vi "Dresden R2R Sputter 03.02.2018 IY24.vi"() -> ()   [LabVIEW 2009] (continued)
                      n13368 = Greater?(x=w19990, y=50) -> (0:w19991:bool)
                      n13369 = local read "Cnt_Right_slow_di"() -> (w19993:bool)
                      n13370 = case shown="True" w19991 {
                        frame #0 {
                        }
                        frame #1 {
                          n13371 = local write "Semi"(TRUE ("Semi")) -> ()
                          n13372 = local write "Error Message"("\nPlease check Left Slow Sensor\nconnections." ("Error Message")) -> ()
                        }
                      }
                      n13373 = case shown="True" w19993 {
                        tunnel: [TRUE ("Cnt_Left_slow_do") FALSE ("Cnt_Left_slow_do")] -> w19989
                        frame #0 {
                        }
                        frame #1 {
                          n13374 = local write "Cnt_Right_slow_do"(FALSE ("Cnt_Left_slow_do")) -> ()
                          n13375 = Wait Until Next ms Multiple(millisecond multiple=u32 200) -> ()  [unwired: 1 out]
                        }
                      }
                      n13376 = local read "Semi"() -> (w19988:bool)
                      n13377 = Or(x=w19989, y=w19988) -> (x .or. y?=w19987:bool)
                    }
                  }
                  frame #2 {
                    n13378 = while {
                      i -> [w20003]
                      stop <- w20000 stop-if-true
                      n13379 = Greater?(x=w20003, y=50) -> (0:w20004:bool)
                      n13380 = local read "Cnt_Right_limit_di"() -> (w20006:bool)
                      n13381 = case shown="True" w20004 {
                        frame #0 {
                        }
                        frame #1 {
                          n13382 = local write "Semi"(TRUE ("Semi")) -> ()
                          n13383 = local write "Error Message"("\nPlease check Left Limit Sensor\n connections." ("Error Message")) -> ()
                        }
                      }
                      n13384 = case shown="True" w20006 {
                        tunnel: [TRUE ("Cnt_Left_slow_do") FALSE ("Cnt_Left_slow_do")] -> w20002
                        frame #0 {
                        }
                        frame #1 {
                          n13385 = local write "Cnt_Right_limit_do"(FALSE ("Cnt_Left_slow_do")) -> ()
                          n13386 = Wait Until Next ms Multiple(millisecond multiple=u32 200) -> ()  [unwired: 1 out]
                        }
                      }
                      n13387 = local read "Semi"() -> (w20001:bool)
                      n13388 = Or(x=w20002, y=w20001) -> (x .or. y?=w20000:bool)
                    }
                  }
                  frame #3 {
                    n13389 = local read "Semi"() -> (w20013:bool)
                    n13390 = case shown="False" w20013 {
                      frame #0 {
                        n13391 = local write "CH1_2trns_12"(TRUE ("CH1_2trns_11")) -> ()
                        n13392 = Wait (ms)(milliseconds to wait=u32 500) -> ()  [unwired: 1 out]
                      }
                      frame #1 {
                      }
                    }
                  }
                }
              }
              frame #1 {
              }
            }
          }
          frame #17 {
            # "SET CASSETTE SERVO  SPEED 100"
            n13393 = local read "Semi"() -> (w20016:bool)
            n13394 = case shown="False" w20016 {
              frame #0 {
                n13395 = stacked-sequence {
                  frame #0 {
                    n13396 = while {
                      i -> [w20023]
                      stop <- w20019 stop-if-true
                      n13397 = local read "Ch2_Right_slow_di"() -> (w20017:bool)
                      n13398 = Greater?(x=w20023, y=1500) -> (0:w20022:bool)
                      n13399 = case shown="True" w20022 {
                        frame #0 {
                        }
                        frame #1 {
                          n13400 = local write "Semi"(TRUE ("Semi")) -> ()
                          n13401 = local write "Error Message"("Transfer process was cancelled.\nPlease check Casette & Sensor\nconnections." ("Error Message")) -> ()
                        }
                      }
                      n13402 = case shown="False" w20017 {
                        tunnel: [FALSE TRUE] -> w20020
                        frame #0 {
                          n13403 = Wait Until Next ms Multiple(millisecond multiple=u32 200) -> ()  [unwired: 1 out]
                        }
                        frame #1 {
                        }
                      }
                      n13404 = local read "Semi"() -> (w20018:bool)
                      n13405 = Or(x=w20020, y=w20018) -> (x .or. y?=w20019:bool)
                    }
                  }
                  frame #1 {
                    n13406 = disable-structure shown="Disabled" {
                      frame #0 {
                        n13407 = while {
                          i -> [w20038]
                          stop <- w20034 stop-if-true
                          n13408 = local read "Counter_read_data"() -> (w20031:i16)
                          n13409 = Greater?(x=w20038, y=5000) -> (0:w20037:bool)
                          n13410 = case shown="True" w20037 {
                            frame #0 {
                            }
                            frame #1 {
                              n13411 = local write "Semi"(TRUE ("Semi")) -> ()
                            }
                          }
                          n13412 = In Range and Coerce(upper limit=i16 1990, x=w20031, lower limit=i16 1980 ("upper limit")) -> (In Range?=w20029:bool)  [unwired: 1 out]
                          n13413 = case shown="True" w20029 {
                            tunnel: [FALSE TRUE] -> w20035
                            frame #0 {
                              n13414 = Wait Until Next ms Multiple(millisecond multiple=u32 200) -> ()  [unwired: 1 out]
                            }
                            frame #1 {
                            }
                          }
                          n13415 = local read "Semi"() -> (w20033:bool)
                          n13416 = Or(x=w20035, y=w20033) -> (x .or. y?=w20034:bool)
                        }
                      }
                      frame #1 {
                      }
                    }
                  }
                  frame #2 {
                    n13417 = local read "Semi"() -> (w20043:bool)
                    n13418 = case shown="False" w20043 {
                      frame #0 {
                        n13419 = local write "Cassette_servo_speed_value"(u16 100 ("Cassette_servo_speed_value")) -> ()
                      }
                      frame #1 {
                      }
                    }
                  }
                  frame #3 {
                    n13420 = local read "Semi"() -> (w20045:bool)
                    n13421 = case shown="False" w20045 {
                      frame #0 {
                        n13422 = Wait (ms)(milliseconds to wait=u32 200 ("millisecond multiple")) -> ()  [unwired: 1 out]
                      }
                      frame #1 {
                      }
                    }
                  }
                  frame #4 {
                    n13423 = local read "Semi"() -> (w20047:bool)
                    n13424 = case shown="False" w20047 {
                      frame #0 {
                        n13425 = local write "Cassette_servo_speed_auto_set"(TRUE ("Cassette_servo_speed_auto_set")) -> ()
                      }
                      frame #1 {
                      }
                    }
                  }
                  frame #5 {
                    n13426 = local read "Semi"() -> (w20049:bool)
                    n13427 = case shown="False" w20049 {
                      frame #0 {
                        n13428 = Wait (ms)(milliseconds to wait=u32 200 ("millisecond multiple")) -> ()  [unwired: 1 out]
                      }
                      frame #1 {
                      }
                    }
                  }
                  frame #6 {
                    n13429 = while {
                      i -> [w20054]
                      stop <- w20051 stop-if-true
                      n13430 = Greater?(x=w20054, y=50) -> (0:w20055:bool)
                      n13431 = local read "Cnt_Right_slow_di"() -> (w20057:bool)
                      n13432 = case shown="True" w20055 {
                        frame #0 {
                        }
                        frame #1 {
                          n13433 = local write "Semi"(TRUE ("Semi")) -> ()
                          n13434 = local write "Error Message"("\nPlease check connections." ("Error Message")) -> ()
                        }
                      }
                      n13435 = case shown="False" w20057 {
                        tunnel: [FALSE ("Cnt_Left_slow_do") TRUE ("Cnt_Left_slow_do")] -> w20053
                        frame #0 {
                          n13436 = local write "Cnt_Right_slow_do"(TRUE ("Cnt_Left_slow_do")) -> ()
                          n13437 = Wait Until Next ms Multiple(millisecond multiple=u32 200) -> ()  [unwired: 1 out]
                        }
                        frame #1 {
                        }
                      }
                      n13438 = local read "Semi"() -> (w20052:bool)
                      n13439 = Or(x=w20053, y=w20052) -> (x .or. y?=w20051:bool)
                    }
                  }
                  frame #7 {
                    n13440 = local read "Semi"() -> (w20064:bool)
                    n13441 = case shown="False" w20064 {
                      frame #0 {
                        n13442 = local write "CH1_2trns_12"(TRUE ("CH1_2trns_11")) -> ()
                        n13443 = Wait (ms)(milliseconds to wait=u32 500) -> ()  [unwired: 1 out]
                      }
                      frame #1 {
                      }
                    }
                  }
                }
              }
              frame #1 {
              }
            }
          }
          frame #18 {
            # "CASETTE STOP AND FIX"
            n13444 = local read "Semi"() -> (w20067:bool)
            n13445 = case shown="False" w20067 {
              frame #0 {
                n13446 = stacked-sequence {
                  frame #0 {
                    # "Center Casette stop"
                    n13447 = local read "Semi"() -> (w20068:bool)
                    n13448 = case shown="False" w20068 {
                      frame #0 {
                        n13449 = stacked-sequence {
                          frame #0 {
                            n13450 = while {
                              i -> [w20075]
                              stop <- w20070 stop-if-true
                              n13451 = local read "Ch2_Right_limit_di"() -> (w20069:bool)
                              n13452 = Greater?(x=w20075, y=600) -> (0:w20073:bool)
                              n13453 = case shown="True" w20073 {
                                frame #0 {
                                }
                                frame #1 {
                                n13454 = local write "Semi"(TRUE ("Semi")) -> ()
                                n13455 = local write "Error Message"("Transfer process was cancelled.\nPlease check Casette connections." ("Error Message")) -> ()
                                }
                              }
                              n13456 = case shown="False" w20069 {
                                tunnel: [FALSE TRUE] -> w20072
                                frame #0 {
                                n13457 = Wait Until Next ms Multiple(millisecond multiple=u32 200) -> ()  [unwired: 1 out]
                                }
                                frame #1 {
                                }
                              }
                              n13458 = local read "Semi"() -> (w20071:bool)
                              n13459 = Or(x=w20072, y=w20071) -> (x .or. y?=w20070:bool)
                            }
                          }
                          frame #1 {
                            n13460 = disable-structure shown="Disabled" {
                              frame #0 {
                                n13461 = while {
                                i -> [w20090]
                                stop <- w20085 stop-if-true
                                n13462 = local read "Counter_read_data"() -> (w20082:i16)
                                n13463 = Greater?(x=w20090, y=5000) -> (0:w20088:bool)
                                n13464 = case shown="True" w20088 {
                                frame #0 {
                                }
                                frame #1 {
                                n13465 = local write "Semi"(TRUE ("Semi")) -> ()
                                n13466 = local write "Error Message"("Transfer process was cancelled.\nPlease check Casette connections." ("Error Message")) -> ()
                                }
                                }
                                n13467 = In Range and Coerce(upper limit=i16 2209, x=w20082, lower limit=i16 2199 ("upper limit")) -> (In Range?=w20081:bool)  [unwired: 1 out]
                                n13468 = case shown="True" w20081 {
                                tunnel: [FALSE TRUE] -> w20087
                                frame #0 {
                                }
                                frame #1 {
                                n13469 = Wait Until Next ms Multiple(millisecond multiple=u32 500) -> ()  [unwired: 1 out]
                                }
                                }
                                n13470 = local read "Semi"() -> (w20086:bool)
                                n13471 = Or(x=w20087, y=w20086) -> (x .or. y?=w20085:bool)
                                }
                              }
                              frame #1 {
                              }
                            }
                          }
                          frame #2 {
                            n13472 = while {
                              i -> [w20102]
                              stop <- w20097 stop-if-true
                              n13473 = local read "Casette_servo_start/stop_di"() -> (w20096:bool)
                              n13474 = Greater?(x=w20102, y=50) -> (0:w20100:bool)
                              n13475 = case shown="True" w20100 {
                                frame #0 {
                                }
                                frame #1 {
                                n13476 = local write "Semi"(TRUE ("Semi")) -> ()
                                n13477 = local write "Error Message"("Transfer process was cancelled.\nPlease check Casette connections." ("Error Message")) -> ()
                                }
                              }
                              n13478 = case shown="True" w20096 {
                                tunnel: [TRUE FALSE] -> w20099
                                frame #0 {
                                }
                                frame #1 {
                                n13479 = Wait Until Next ms Multiple(millisecond multiple=u32 200) -> ()  [unwired: 1 out]
                                n13480 = local write "Casette_servo_start/stop_do"(FALSE ("Casette_servo_start/stop_di")) -> ()
                                }
                              }
                              n13481 = local read "Semi"() -> (w20098:bool)
                              n13482 = Or(x=w20099, y=w20098) -> (x .or. y?=w20097:bool)
                            }
                          }
                          frame #3 {
                            n13483 = local read "Semi"() -> (w20109:bool)
                            n13484 = case shown="False" w20109 {
                              frame #0 {
                                n13485 = Wait (ms)(milliseconds to wait=u32 200) -> ()  [unwired: 1 out]
                              }
                              frame #1 {
                              }
                            }
                          }
                          frame #4 {
                            n13486 = local read "Semi"() -> (w20111:bool)
                            n13487 = case shown="False" w20111 {
                              frame #0 {
                                n13488 = local write "Cassette_servo_speed_value"(u16 0 ("Cassette_servo_speed_value")) -> ()
                              }
                              frame #1 {
                              }
                            }
                          }
                          frame #5 {
                            n13489 = local read "Semi"() -> (w20113:bool)
                            n13490 = case shown="False" w20113 {
                              frame #0 {
                                n13491 = Wait (ms)(milliseconds to wait=u32 200) -> ()  [unwired: 1 out]
                              }
                              frame #1 {
                              }
                            }
                          }
                          frame #6 {
                            n13492 = local read "Semi"() -> (w20115:bool)
                            n13493 = case shown="False" w20115 {
                              frame #0 {
                                n13494 = local write "Cassette_servo_speed_auto_set"(TRUE ("Cassette_servo_speed_auto_set")) -> ()
                              }
                              frame #1 {
                              }
                            }
                          }
                          frame #7 {
                            n13495 = local read "Semi"() -> (w20117:bool)
                            n13496 = case shown="False" w20117 {
                              frame #0 {
                                n13497 = Wait (ms)(milliseconds to wait=u32 200) -> ()  [unwired: 1 out]
                              }
                              frame #1 {
                              }
                            }
                          }
                          frame #8 {
                            n13498 = local read "Semi"() -> (w20119:bool)
                            n13499 = case shown="False" w20119 {
                              frame #0 {
                                n13500 = local write "CH1_2trns_13"(TRUE ("CH1_2trns_9")) -> ()
                                n13501 = Wait (ms)(milliseconds to wait=u32 500) -> ()  [unwired: 1 out]
                              }
                              frame #1 {
                              }
                            }
                          }
                        }
                      }
                      frame #1 {
                      }
                    }
                  }
                  frame #1 {
                    # "CASETTE FIX DOWN CH2"
                    n13502 = local read "Semi"() -> (w20122:bool)
                    n13503 = case shown="False" w20122 {
                      frame #0 {
                        n13504 = stacked-sequence {
                          frame #0 {
                            n13505 = local read "Semi"() -> (w20123:bool)
                            n13506 = case shown="False" w20123 {
                              frame #0 {
                                n13507 = while {
                                i -> [w20130]
                                stop <- w20125 stop-if-true
                                n13508 = Greater?(x=w20130, y=50) -> (0:w20128:bool)
                                n13509 = local read "Ch2_Cst_fix_down_di"() -> (w20124:bool)
                                n13510 = case shown="True" w20128 {
                                frame #0 {
                                }
                                frame #1 {
                                n13511 = local write "Semi"(TRUE ("Semi")) -> ()
                                n13512 = local write "Error Message"("Up/Down positions could not reach\nthe down position.\nPlease check connections." ("Error Message")) -> ()
                                }
                                }
                                n13513 = case shown="False" w20124 {
                                tunnel: [FALSE TRUE] -> w20127
                                frame #0 {
                                n13514 = Wait Until Next ms Multiple(millisecond multiple=u32 200) -> ()  [unwired: 1 out]
                                n13515 = local write "Ch2_Cst_fix_do"(TRUE ("Ch1_pet_cool_up_do")) -> ()
                                }
                                frame #1 {
                                }
                                }
                                n13516 = local read "Semi"() -> (w20126:bool)
                                n13517 = Or(x=w20127, y=w20126) -> (x .or. y?=w20125:bool)
                                }
                              }
                              frame #1 {
                              }
                            }
                          }
                          frame #1 {
                            n13518 = local read "Semi"() -> (w20137:bool)
                            n13519 = case shown="False" w20137 {
                              frame #0 {
                                n13520 = local write "CH1_2trns_14"(TRUE ("CH1_2trns_9")) -> ()
                                n13521 = Wait (ms)(milliseconds to wait=u32 500) -> ()  [unwired: 1 out]
                              }
                              frame #1 {
                              }
                            }
                          }
                        }
                      }
                      frame #1 {
                      }
                    }
                  }
                  frame #2 {
                    n13522 = local read "Semi"() -> (w20140:bool)
                    n13523 = case shown="False" w20140 {
                      frame #0 {
                        n13524 = stacked-sequence {
                          frame #0 {
                            n13525 = local read "Semi"() -> (w20141:bool)
                            n13526 = case shown="False" w20141 {
                              frame #0 {
                                n13527 = while {
                                i -> [w20148]
                                stop <- w20143 stop-if-true
                                n13528 = Greater?(x=w20148, y=50) -> (0:w20146:bool)
                                n13529 = local read "Ch2_trns_gv_bp2_di"() -> (w20142:bool)
                                n13530 = case shown="True" w20146 {
                                frame #0 {
                                }
                                frame #1 {
                                n13531 = local write "Semi"(TRUE ("Semi")) -> ()
                                n13532 = local write "Error Message"("Transfer process was cancelled.\nPlease check CH1-Trns-GV connections." ("Error Message")) -> ()
                                }
                                }
                                n13533 = case shown="True" w20142 {
                                tunnel: [TRUE FALSE] -> w20145
                                frame #0 {
                                }
                                frame #1 {
                                n13534 = Wait Until Next ms Multiple(millisecond multiple=u32 200) -> ()  [unwired: 1 out]
                                n13535 = local write "Ch2_trns_gv_bp2_do"(FALSE ("Ch1_pet_cool_up_do")) -> ()
                                }
                                }
                                n13536 = local read "Semi"() -> (w20144:bool)
                                n13537 = Or(x=w20145, y=w20144) -> (x .or. y?=w20143:bool)
                                }
                              }
                              frame #1 {
                              }
                            }
                          }
                          frame #1 {
                            n13538 = local read "Semi"() -> (w20155:bool)
                            n13539 = case shown="False" w20155 {
                              frame #0 {
                                n13540 = Wait (ms)(milliseconds to wait=u32 500) -> ()  [unwired: 1 out]
                              }
                              frame #1 {
                              }
                            }
                          }
                          frame #2 {
                            n13541 = local read "Semi"() -> (w20157:bool)
                            n13542 = case shown="False" w20157 {
                              frame #0 {
                                n13543 = while {
                                i -> [w20164]
                                stop <- w20159 stop-if-true
                                n13544 = Greater?(x=w20164, y=50) -> (0:w20162:bool)
                                n13545 = local read "Ch3_Trns_gv_bp_di"() -> (w20158:bool)
                                n13546 = case shown="True" w20162 {
                                frame #0 {
                                }
                                frame #1 {
                                n13547 = local write "Semi"(TRUE ("Semi")) -> ()
                                n13548 = local write "Error Message"("Transfer process was cancelled.\nPlease check CH1-Trns-GV connections." ("Error Message")) -> ()
                                }
                                }
                                n13549 = case shown="True" w20158 {
                                tunnel: [TRUE FALSE] -> w20161
                                frame #0 {
                                }
                                frame #1 {
                                n13550 = local write "Ch3_Trns_gv_bp_do"(FALSE ("Ch1_pet_cool_up_do")) -> ()
                                n13551 = Wait Until Next ms Multiple(millisecond multiple=u32 200) -> ()  [unwired: 1 out]
                                }
                                }
                                n13552 = local read "Semi"() -> (w20160:bool)
                                n13553 = Or(x=w20161, y=w20160) -> (x .or. y?=w20159:bool)
                                }
                              }
                              frame #1 {
                              }
                            }
                          }
                          frame #3 {
                            n13554 = local read "Semi"() -> (w20171:bool)
                            n13555 = case shown="False" w20171 {
                              frame #0 {
                                n13556 = Wait (ms)(milliseconds to wait=u32 500) -> ()  [unwired: 1 out]
                              }
                              frame #1 {
                              }
                            }
                          }
                        }
                      }
                      frame #1 {
                      }
                    }
                  }
                  frame #3 {
                    n13557 = local read "Semi"() -> (w20173:bool)
                    n13558 = case shown="False" w20173 {
                      frame #0 {
                        n13559 = stacked-sequence {
                          frame #0 {
                            n13560 = local read "Semi"() -> (w20174:bool)
                            n13561 = case shown="False" w20174 {
                              frame #0 {
                                n13562 = local write "Ch2_Trns_gv_open_do"(FALSE ("Ch1_pet_cool_up_do")) -> ()
                              }
                              frame #1 {
                              }
                            }
                          }
                          frame #1 {
                            n13563 = local read "Semi"() -> (w20176:bool)
                            n13564 = case shown="False" w20176 {
                              frame #0 {
                                n13565 = while {
                                i -> [w20183]
                                stop <- w20178 stop-if-true
                                n13566 = Greater?(x=w20183, y=500) -> (0:w20181:bool)
                                n13567 = local read "Ch2_Trns_gv_close_di"() -> (w20177:bool)
                                n13568 = case shown="True" w20181 {
                                frame #0 {
                                }
                                frame #1 {
                                n13569 = local write "Semi"(TRUE ("Semi")) -> ()
                                n13570 = local write "Error Message"("Transfer process was cancelled.\nPlease check  GV connections." ("Error Message")) -> ()
                                }
                                }
                                n13571 = case shown="False" w20177 {
                                tunnel: [FALSE TRUE] -> w20180
                                frame #0 {
                                n13572 = Wait Until Next ms Multiple(millisecond multiple=u32 200) -> ()  [unwired: 1 out]
                                n13573 = local write "Ch2_Trns_gv_close_do"(TRUE ("Ch1_pet_cool_up_do")) -> ()
                                }
                                frame #1 {
                                }
                                }
                                n13574 = local read "Semi"() -> (w20179:bool)
                                n13575 = Or(x=w20180, y=w20179) -> (x .or. y?=w20178:bool)
                                }
                              }
                              frame #1 {
                              }
                            }
                          }
                          frame #2 {
                            n13576 = local read "Semi"() -> (w20190:bool)
                            n13577 = case shown="False" w20190 {
                              frame #0 {
                                n13578 = local write "CH1_2trns_17"(TRUE ("CH1_2trns_9")) -> ()
                                n13579 = Wait (ms)(milliseconds to wait=u32 500) -> ()  [unwired: 1 out]
                              }
                              frame #1 {
                              }
                            }
                          }
                        }
                      }
                      frame #1 {
                      }
                    }
                  }
                  frame #4 {
                    # "PET COOL DOWN OF CH2"
                    n13580 = local read "Semi"() -> (w20193:bool)
                    n13581 = case shown="False" w20193 {
                      frame #0 {
                        n13582 = stacked-sequence {
                          frame #0 {
                            n13583 = local read "Semi"() -> (w20194:bool)
                            n13584 = case shown="False" w20194 {
                              frame #0 {
                                n13585 = local write "Ch2_Pet_cool_up_do"(FALSE ("Ch1_pet_cool_up_do")) -> ()
                              }
                              frame #1 {
                              }
                            }
                          }
                          frame #1 {
                            n13586 = local read "Semi"() -> (w20196:bool)
                            n13587 = case shown="False" w20196 {
                              frame #0 {
                                n13588 = while {
                                i -> [w20203]
                                stop <- w20198 stop-if-true
                                n13589 = Greater?(x=w20203, y=300) -> (0:w20201:bool)
                                n13590 = case shown="True" w20201 {
                                frame #0 {
                                }
                                frame #1 {
                                n13591 = local write "Semi"(TRUE ("Semi")) -> ()
                                n13592 = local write "Error Message"("SBS Cool Up/Down positions could not reach\nthe down position.\nPlease check connections." ("Error Message")) -> ()
                                }
                                }
                                n13593 = local read "Ch2_Pet_cool_down_di"() -> (w20197:bool)
                                n13594 = case shown="False" w20197 {
                                tunnel: [FALSE TRUE] -> w20200
                                frame #0 {
                                n13595 = Wait Until Next ms Multiple(millisecond multiple=u32 200) -> ()  [unwired: 1 out]
                                n13596 = local write "Ch2_Pet_cool_down_do"(TRUE ("Ch1_pet_cool_up_do")) -> ()
                                }
                                frame #1 {
                                }
                                }
                                n13597 = local read "Semi"() -> (w20199:bool)
                                n13598 = Or(x=w20200, y=w20199) -> (x .or. y?=w20198:bool)
                                }
                              }
                              frame #1 {
                              }
                            }
                          }
                          frame #2 {
                            n13599 = local read "Semi"() -> (w20210:bool)
                            n13600 = case shown="False" w20210 {
                              frame #0 {
                                n13601 = local write "CH1_2trns_15"(TRUE ("CH1_2trns_9")) -> ()
                                n13602 = Wait (ms)(milliseconds to wait=u32 500) -> ()  [unwired: 1 out]
                              }
                              frame #1 {
                              }
                            }
                          }
                        }
                      }
                      frame #1 {
                      }
                    }
                  }
                  frame #5 {
                    # "SRV PIS FOR"
                    n13603 = local read "Semi"() -> (w20213:bool)
                    n13604 = case shown="False" w20213 {
                      frame #0 {
                        n13605 = stacked-sequence {
                          frame #0 {
                            n13606 = local read "Semi"() -> (w20214:bool)
                            n13607 = case shown="False" w20214 {
                              frame #0 {
                                n13608 = local write "Ch2_SRV1_PIST_Back_do"(FALSE ("Ch1_pet_cool_up_do")) -> ()
                              }
                              frame #1 {
                              }
                            }
                          }
                          frame #1 {
                            n13609 = local read "Semi"() -> (w20216:bool)
                            n13610 = case shown="False" w20216 {
                              frame #0 {
                                n13611 = while {
                                i -> [w20223]
                                stop <- w20218 stop-if-true
                                n13612 = Greater?(x=w20223, y=100) -> (0:w20221:bool)
                                n13613 = local read "Ch2_SRV1_PIST For_di"() -> (w20217:bool)
                                n13614 = case shown="True" w20221 {
                                frame #0 {
                                }
                                frame #1 {
                                n13615 = local write "Semi"(TRUE ("Semi")) -> ()
                                n13616 = local write "Error Message"("For/Back positions could not reach\nthe forward position.\nPlease check connections." ("Error Message")) -> ()
                                }
                                }
                                n13617 = case shown="False" w20217 {
                                tunnel: [FALSE TRUE] -> w20220
                                frame #0 {
                                n13618 = Wait Until Next ms Multiple(millisecond multiple=u32 200) -> ()  [unwired: 1 out]
                                n13619 = local write "Ch2_SRV1_PIST For_do"(TRUE ("Ch1_pet_cool_up_do")) -> ()
                                }
                                frame #1 {
                                }
                                }
                                n13620 = local read "Semi"() -> (w20219:bool)
                                n13621 = Or(x=w20220, y=w20219) -> (x .or. y?=w20218:bool)
                                }
                              }
                              frame #1 {
                              }
                            }
                          }
                          frame #2 {
                            n13622 = local read "Semi"() -> (w20230:bool)
                            n13623 = case shown="False" w20230 {
                              frame #0 {
                                n13624 = local write "CH1_2trns_16"(TRUE ("CH1_2trns_9")) -> ()
                                n13625 = Wait (ms)(milliseconds to wait=u32 500) -> ()  [unwired: 1 out]
                              }
                              frame #1 {
                              }
                            }
                          }
                        }
                      }
                      frame #1 {
                      }
                    }
                  }
                }
              }
              frame #1 {
              }
            }
          }
          frame #19 {
            # "Sensors deactive"
            n13626 = local read "Semi"() -> (w20233:bool)
            n13627 = case shown="False" w20233 {
              frame #0 {
                n13628 = stacked-sequence {
                  frame #0 {
                    n13629 = local read "Semi"() -> (w20234:bool)
                    n13630 = case shown="False" w20234 {
                      frame #0 {
                        n13631 = while {
                          i -> [w20237]
                          stop <- w20238 stop-if-true
                          n13632 = Greater?(x=w20237, y=50) -> (0:w20235:bool)
                          n13633 = local read "Cnt_Right_slow_di"() -> (w20241:bool)
                          n13634 = case shown="True" w20235 {
                            frame #0 {
                            }
                            frame #1 {
                              n13635 = local write "Semi"(TRUE ("Semi")) -> ()
                              n13636 = local write "Error Message"("Transfer process was\ncancelled.Please check right slow sensor." ("Error Message")) -> ()
                            }
                          }
                          n13637 = case shown="False" w20241 {
                            tunnel: [FALSE ("Ch1_pet_cool_up_do") TRUE ("Ch1_pet_cool_up_do")] -> w20240
                            frame #0 {
                              n13638 = Wait Until Next ms Multiple(millisecond multiple=u32 200) -> ()  [unwired: 1 out]
                              n13639 = local write "Cnt_Right_slow_do"(TRUE ("Ch1_pet_cool_up_do")) -> ()
                            }
                            frame #1 {
                            }
                          }
                          n13640 = local read "Semi"() -> (w20239:bool)
                          n13641 = Or(x=w20240, y=w20239) -> (x .or. y?=w20238:bool)
                        }
                      }
                      frame #1 {
                      }
                    }
                  }
                  frame #1 {
                    n13642 = local read "Semi"() -> (w20248:bool)
                    n13643 = case shown="False" w20248 {
                      frame #0 {
                        n13644 = while {
                          i -> [w20251]
                          stop <- w20252 stop-if-true
                          n13645 = Greater?(x=w20251, y=50) -> (0:w20249:bool)
                          n13646 = local read "Cnt_Right_limit_di"() -> (w20255:bool)
                          n13647 = case shown="True" w20249 {
                            frame #0 {
                            }
                            frame #1 {
                              n13648 = local write "Semi"(TRUE ("Semi")) -> ()
                              n13649 = local write "Error Message"("Transfer process was\ncancelled.Please check right limit sensor." ("Error Message")) -> ()
                            }
                          }
                          n13650 = case shown="False" w20255 {
                            tunnel: [FALSE ("Ch1_pet_cool_up_do") TRUE ("Ch1_pet_cool_up_do")] -> w20254
                            frame #0 {
                              n13651 = Wait Until Next ms Multiple(millisecond multiple=u32 200) -> ()  [unwired: 1 out]
                              n13652 = local write "Cnt_Right_limit_do"(TRUE ("Ch1_pet_cool_up_do")) -> ()
                            }
                            frame #1 {
                            }
                          }
                          n13653 = local read "Semi"() -> (w20253:bool)
                          n13654 = Or(x=w20254, y=w20253) -> (x .or. y?=w20252:bool)
                        }
                      }
                      frame #1 {
                      }
                    }
                  }
                  frame #2 {
                    n13655 = local read "Semi"() -> (w20262:bool)
                    n13656 = case shown="False" w20262 {
                      frame #0 {
                        n13657 = while {
                          i -> [w20265]
                          stop <- w20266 stop-if-true
                          n13658 = Greater?(x=w20265, y=50) -> (0:w20263:bool)
                          n13659 = local read "Cnt_Left_slow_di"() -> (w20269:bool)
                          n13660 = case shown="True" w20263 {
                            frame #0 {
                            }
                            frame #1 {
                              n13661 = local write "Semi"(TRUE ("Semi")) -> ()
                              n13662 = local write "Error Message"("Transfer process was\ncancelled.Please check left slow sensor." ("Error Message")) -> ()
                            }
                          }
                          n13663 = case shown="False" w20269 {
                            tunnel: [FALSE ("Ch1_pet_cool_up_do") TRUE ("Ch1_pet_cool_up_do")] -> w20268
                            frame #0 {
                              n13664 = Wait Until Next ms Multiple(millisecond multiple=u32 200) -> ()  [unwired: 1 out]
                              n13665 = local write "Cnt_Left_slow_do"(TRUE ("Ch1_pet_cool_up_do")) -> ()
                            }
                            frame #1 {
                            }
                          }
                          n13666 = local read "Semi"() -> (w20267:bool)
                          n13667 = Or(x=w20268, y=w20267) -> (x .or. y?=w20266:bool)
                        }
                      }
                      frame #1 {
                      }
                    }
                  }
                  frame #3 {
                    n13668 = local read "Semi"() -> (w20276:bool)
                    n13669 = case shown="False" w20276 {
                      frame #0 {
                        n13670 = while {
                          i -> [w20279]
                          stop <- w20280 stop-if-true
                          n13671 = Greater?(x=w20279, y=50) -> (0:w20277:bool)
                          n13672 = local read "Cnt_Left_limit_di"() -> (w20283:bool)
                          n13673 = case shown="True" w20277 {
                            frame #0 {
                            }
                            frame #1 {
                              n13674 = local write "Semi"(TRUE ("Semi")) -> ()
                              n13675 = local write "Error Message"("Transfer process was\ncancelled.Please check left limit sensor." ("Error Message")) -> ()
                            }
                          }
                          n13676 = case shown="False" w20283 {
                            tunnel: [FALSE ("Ch1_pet_cool_up_do") TRUE ("Ch1_pet_cool_up_do")] -> w20282
                            frame #0 {
                              n13677 = Wait Until Next ms Multiple(millisecond multiple=u32 200) -> ()  [unwired: 1 out]
                              n13678 = local write "Cnt_Left_limit_do"(TRUE ("Ch1_pet_cool_up_do")) -> ()
                            }
                            frame #1 {
                            }
                          }
                          n13679 = local read "Semi"() -> (w20281:bool)